vi "Dresden R2R Sputter 03.02.2018 IY24.vi"() -> ()   [LabVIEW 2009] (continued)
        n23727 = local write "R Single DC Step4 Coating Power"(w29188) -> ()
        n23728 = local write "R Single RF Step2 Coating Power"(w29146) -> ()
        n23729 = local write "R Single RF Interval length"(w29148) -> ()
        n23730 = case shown="2" w29281 {
          frame #0 {
          }
          frame #1 {
            n23731 = local write "R_Recipe_type_selection"(enum32{"Single Recipe", "Combination Sputter"}."Single Recipe" ("R_Recipe_type_selection")) -> ()
          }
          frame #2 {
            n23732 = local write "R_Recipe_type_selection"(enum32{"Single Recipe", "Combination Sputter"}."Combination Sputter" ("R_Recipe_type_selection")) -> ()
          }
        }
        n23733 = local write "R Single RF Step3 Coating Power"(w29144) -> ()
        n23734 = local write "R Web speed(cm/min)"(w29259) -> ()
        n23735 = Boolean Array To Number(Boolean array=w29296) -> (number=w29295:u32)
        n23736 = local write "R Single RF Step4 Coating Power"(w29142) -> ()
        n23737 = local write "R Maximum diameter"(w29261) -> ()
        n23738 = case shown="2" w29348 {
          frame #0 {
          }
          frame #1 {
            n23739 = local write "R_Web_selection"(enum32{"Web", "Other"}."Web" ("R_Web_selection")) -> ()
          }
          frame #2 {
            n23740 = local write "R_Web_selection"(enum32{"Web", "Other"}."Other" ("R_Web_selection")) -> ()
          }
        }
        n23741 = local write "R Minimum diameter"(w29262) -> ()
        n23742 = local write "R_Single Microwave Power"(w28900) -> ()
        n23743 = local write "R Single RF Step5 Coating Power"(w29138) -> ()
        n23744 = local write "R_Single Microwave Time"(w29233) -> ()
        n23745 = local write "R Single Microwave Number"(w29234) -> ()
        n23746 = local write "R _Total_length"(w28935) -> ()
        n23747 = Mantissa & Exponent(0:w29295) -> (2:w29289:dbl)  [unwired: 1 out]
        n23748 = local write "R Tension Value"(w29258) -> ()
        n23749 = local write "R Single RF Ramp down Time"(w29134) -> ()
        n23750 = local write "R Web thicness"(w29260) -> ()
        n23751 = case shown="2" w29300 {
          frame #0 {
          }
          frame #1 {
            n23752 = local write "R_Thickness Selection"(enum32{"Thickness", "Time"}."Thickness" ("R_Thickness Selection")) -> ()
          }
          frame #2 {
            n23753 = local write "R_Thickness Selection"(enum32{"Thickness", "Time"}."Time" ("R_Thickness Selection")) -> ()
          }
        }
        n23754 = case shown="3" w29289 {
          frame #0 {
          }
          frame #1 {
            n23755 = local write "R_Simple_Coating Type Selection"(T3."Microwave Plasma" ("R_Coating Type Selection")) -> ()
          }
          frame #2 {
            n23756 = local write "R_Simple_Coating Type Selection"(T3."DC Sputter" ("R_Coating Type Selection")) -> ()
          }
          frame #3 {
            n23757 = local write "R_Simple_Coating Type Selection"(T3."RF Sputter" ("R_Coating Type Selection")) -> ()
          }
        }
        n23758 = Build Array(FALSE, w28934, w28927) -> (w28931:bool[])
        n23759 = Boolean Array To Number(Boolean array=w28931) -> (number=w28932:u32)
        n23760 = Mantissa & Exponent(0:w28932) -> (2:w28929:dbl)  [unwired: 1 out]
        n23761 = stacked-sequence {
          frame #0 {
            # "Recipe Parameters"
          }
        }
        n23762 = case shown="1" w28929 {
          frame #0 {
          }
          frame #1 {
            n23763 = local write "R_DC_Chamber_selection"(enum32{"Chamber II", "Chamber III"}."Chamber II" ("R_DC_Chamber_selection")) -> ()
          }
          frame #2 {
            n23764 = local write "R_DC_Chamber_selection"(enum32{"Chamber II", "Chamber III"}."Chamber III" ("R_DC_Chamber_selection")) -> ()
          }
        }
      }
    }
    n23765 = case shown="True" "Edit_recipe" {
      frame #0 {
      }
      frame #1 {
        n23766 = call "Dresden Edit Recipe(in).vi"() -> ()  [unwired: 1 in]
      }
    }
    n23767 = case shown="True" "Edit_coating" {
      frame #0 {
      }
      frame #1 {
        n23768 = call "VK-1701Edit Coating.vi"() -> ()  [unwired: 3 in]
      }
    }
    n23769 = case shown="True" "New_recipe" {
      frame #0 {
      }
      frame #1 {
        n23770 = call "Dresden New Recipe(in).vi"() -> ()  [unwired: 2 out]
      }
    }
    n23771 = case shown="True" "New_coating" {
      frame #0 {
      }
      frame #1 {
        n23772 = call "VK-1701New Coating.vi"() -> ()  [unwired: 1 in, 2 out]
      }
    }
    n23773 = case shown="True" "Load_coating" {
      frame #0 {
      }
      frame #1 {
        n23774 = call "VK-1701Load Coating.vi"() -> ("Path Array"=w28844:string[])  [unwired: 1 in, 2 out]
        "Path Array" <- w28844
        n23775 = Array Size(array=w28844) -> (size(s)=w28847:i32)
        n23776 = Increment(x=w28847) -> (x+1=w28848:i32)
        n23777 = Reshape Array(w28844, w28848, w28848) -> (w28849:string[][])
        n23778 = Decrement(x=w28847) -> (x-1=→"Size":i32)
        n23779 = Transpose 2D Array(2D array=w28849) -> (transposed array=w28845:string[][])
        n23780 = property on="Recipe List" class="MCListbox (strict)"("ItemNames"=w28845) -> ()  [unwired: 2 in, 2 out]
      }
    }
    n23781 = local read "Start_coating"() -> (w28837:bool)
    n23782 = case shown="True" w28837 {
      frame #0 {
      }
      frame #1 {
        n23783 = local read "Semi"() -> (w28858:bool)
        n23784 = local read "Recipe_number"() -> (w28851:i32)
        n23785 = local read "Size"() -> (w28855:i32)
        n23786 = Or(x=w28858, y="Coat_int") -> (x .or. y?=w28861:bool)
        n23787 = Increment(x=w28855) -> (x+1=w28856:i32)
        n23788 = feedback #446() -> (w28852:i32)  [unwired: 1 in]
        n23789 = Equal?(x=w28851, y=w28856) -> (x = y?=w28857:bool)
        n23790 = Greater?(x=w28851, y=w28852) -> (0:w28853:bool)
        n23791 = Or(x=w28853, y=w28857) -> (x .or. y?=w28850:bool)
        n23792 = Build Array(FALSE, w28861, w28850) -> (w28863:bool[])
        n23793 = Boolean Array To Number(Boolean array=w28863) -> (number=w28862:u32)
        n23794 = Mantissa & Exponent(0:w28862) -> (2:w28854:dbl)  [unwired: 1 out]
        n23795 = case shown="2" w28854 {
          frame #0 {
            n23796 = stacked-sequence {
              tunnel: [w28870] -> w28864
              frame #0 {
                n23797 = local read "Recipe_number"() -> (w28872:i32)
                n23798 = local read "Size"() -> (w28873:i32)
                n23799 = Increment(x=w28873) -> (x+1=w28871:i32)
                n23800 = Equal?(x=w28872, y=w28871) -> (x = y?=w28870:bool)
              }
            }
            n23801 = case shown="False" w28864 {
              frame #0 {
                n23802 = property on="Recipe List" class="MCListbox (strict)"() -> ("ItemNames"=w28866:string[][])  [unwired: 2 in, 2 out]
                n23803 = local read "Recipe_number"() -> (w28867:i32)
                n23804 = Replace Array Subset(array=w28866, new element="Running" ("new element/subarray"), index (row)=w28867, index (col)=1 ("Column")) -> (w28865:string[][])
                n23805 = property on="Recipe List" class="MCListbox (strict)"("ItemNames"=w28865) -> ()  [unwired: 2 in, 2 out]
              }
              frame #1 {
              }
            }
          }
          frame #1 {
            n23806 = local read "Recipe_number"() -> (w28874:i32)
            n23807 = property on="Recipe List" class="MCListbox (strict)"() -> ("ItemNames"=w28876:string[][])  [unwired: 2 in, 2 out]
            n23808 = Replace Array Subset(array=w28876, new element="Not Completed !" ("new element/subarray"), index (row)=w28874, index (col)=1 ("Column")) -> (w28875:string[][])
            n23809 = property on="Recipe List" class="MCListbox (strict)"("ItemNames"=w28875) -> ()  [unwired: 2 in, 2 out]
          }
          frame #2 {
            n23810 = property on="Recipe List" class="MCListbox (strict)"() -> ("ItemNames"=w28880:string[][])  [unwired: 2 in, 2 out]
            n23811 = stacked-sequence {
              tunnel: [_ w28890] -> w28884
              frame #0 {
                n23812 = Wait (ms)(milliseconds to wait=u32 1000) -> ()  [unwired: 1 out]
              }
              frame #1 {
                n23813 = local read "Size"() -> (w28893:i32)
                n23814 = Less?(x=w28893, y=1) -> (x < y?=w28895:bool)
                n23815 = case shown="True" w28895 {
                  tunnel: [w28897 w28898] -> w28891
                  tunnel: w28893 -> [w28896 w28898]
                  frame #0 {
                    n23816 = Increment(x=w28896) -> (x+1=w28897:i32)
                  }
                  frame #1 {
                  }
                }
                n23817 = local read "Recipe_number"() -> (w28892:i32)
                n23818 = Equal?(x=w28892, y=w28891) -> (x = y?=w28890:bool)
              }
            }
            n23819 = case shown="False" w28884 {
              tunnel: [w28885 w28887] -> w28881
              frame #0 {
                n23820 = local read "Recipe_number"() -> (w28886:i32)
                n23821 = Decrement(x=w28886) -> (x-1=w28885:i32)
              }
              frame #1 {
                n23822 = local read "Recipe_number"() -> (w28888:i32)
                n23823 = Decrement(x=w28888) -> (x-1=w28887:i32)
              }
            }
            n23824 = Replace Array Subset(array=w28880, new element="Done" ("new element/subarray"), index (row)=w28881, index (col)=1 ("Column")) -> (w28879:string[][])
            n23825 = property on="Recipe List" class="MCListbox (strict)"("ItemNames"=w28879) -> ()  [unwired: 2 in, 2 out]
          }
        }
      }
    }
  }
  n23826 = while {
    stop <- FALSE stop-if-true
    n23827 = Wait Until Next ms Multiple(millisecond multiple=u32 300) -> ()  [unwired: 1 out]
    n23828 = Compound Arithmetic op=OR("Start_Coating_MW", "Start_Coating_Ch2", "Start_Coating_Ch3", "Start_Coating_Ch4") -> (w29415:bool)
    n23829 = case shown="True" w29415 {
      frame #0 {
      }
      frame #1 {
        n23830 = local write "Start_coating"(TRUE ("Start_coating")) -> ()
      }
    }
  }
  n23831 = while {
    stop <- FALSE stop-if-true
    n23832 = Wait Until Next ms Multiple(millisecond multiple=u32 300) -> ()  [unwired: 1 out]
    n23833 = case shown="True" "Start_coating" {
      frame #0 {
      }
      frame #1 {
        n23834 = while {
          i -> [w29428]
          stop <- w29422 stop-if-true
          n23835 = Wait Until Next ms Multiple(millisecond multiple=u32 300) -> ()  [unwired: 1 out]
          n23836 = local read "Path Array"() -> (w29427:string[])
          n23837 = Index Array(array=w29427, index=w29428) -> (element=w29425:string)
          "Path" <- w29425
          n23838 = Not Equal?(x="", y=w29425) -> (x != y?=w29424:bool)
          n23839 = case shown="True" w29424 {
            tunnel: [TRUE w29431] -> w29422
            frame #0 {
              w29429 = FALSE
              n23840 = local write "Start_Coating_MW"(w29429) -> ()
              n23841 = local write "Start_coating"(w29429) -> ()
              n23842 = local write "Start_Coating_Ch2"(w29429) -> ()
              n23843 = local write "Start_Coating_Ch3"(w29429) -> ()
              n23844 = local write "Start_Coating_Ch4"(w29429) -> ()
            }
            frame #1 {
              n23845 = stacked-sequence {
                tunnel: [FALSE _] -> w29431
                frame #0 {
                  # "All Recipe Parameters close &set zero"
                  n23846 = stacked-sequence {
                    frame #0 {
                      w29435 = FALSE ("Single_ Target_clean_cancel")
                      w29436 = FALSE ("Visible")
                      w29434 = TRUE ("Clean_MW_Coating")
                      w29437 = FALSE ("Cnt_Right_limit_do")
                      w29440 = FALSE ("R Single RF Ramp down")
                      w29441 = FALSE ("R Cmb Ch3 DC Target Clean Power Active")
                      w29442 = 0.0 ("R Cmb Ch2 Step4 Coating Power")
                      w29438 = 0.0 ("Preheating Temperature")
                      w29439 = "" ("Recipe Name :")
                      n23847 = local write "Substrate Material"(w29439) -> ()
                      n23848 = local write "R Cmb Ch2 Target material"(w29439) -> ()
                      n23849 = local write "R Single DC Target material"(w29439) -> ()
                      n23850 = local write "R Cmb Ch3 Target material"(w29439) -> ()
                      n23851 = local write "R Single RF Target material"(w29439) -> ()
                      n23852 = local write "Recipe Name"(w29439) -> ()
                      n23853 = property on="Process_tab_sputter 3" class="TabCtl (strict)"("Visible"=w29436) -> ()  [unwired: 2 in, 2 out]
                      n23854 = property on="Sputter_tab 3" class="TabCtl (strict)"("Visible"=w29436) -> ()  [unwired: 2 in, 2 out]
                      n23855 = property on="Process_tab_sputter" class="TabCtl (strict)"("Visible"=w29436) -> ()  [unwired: 2 in, 2 out]
                      n23856 = property on="Sputter_tab" class="TabCtl (strict)"("Visible"=w29436) -> ()  [unwired: 2 in, 2 out]
                      n23857 = property on="Sputter_tab 2" class="TabCtl (strict)"("Visible"=w29436) -> ()  [unwired: 2 in, 2 out]
                      n23858 = local write "R_Single Microwave Power"(w29438) -> ()
                      n23859 = local write "R_Single Microwave Time"(w29438) -> ()
                      n23860 = local write "R Single DC Ignition Power"(w29438) -> ()
                      n23861 = local write "R Single DC Target Clean Power"(w29438) -> ()
                      n23862 = local write "R Single DC Target Clean Time"(w29438) -> ()
                      n23863 = local write "R Single RF Ramp up Time"(w29438) -> ()
                      n23864 = local write "R Single RF Ignition Power"(w29438) -> ()
                      n23865 = local write "R Single RF Target Clean Power"(w29438) -> ()
                      n23866 = local write "R Single RF Target Clean Time"(w29438) -> ()
                      n23867 = local write "R Single RF Ramp down Time"(w29438) -> ()
                      n23868 = local write "R Cmb Ch2 DC Ignition Power"(w29438) -> ()
                      n23869 = local write "R Cmb Ch2 DC Target Clean Power"(w29438) -> ()
                      n23870 = local write "R Cmb Ch2 DC Target Clean Time"(w29438) -> ()
                      n23871 = local write "R Cmb Ch2 Step1 Coating Power"(w29438) -> ()
                      n23872 = local write "R Cmb Ch2 Step2 Coating Power"(w29438) -> ()
                      n23873 = local write "R Cmb Ch2 Step3 Coating Power"(w29438) -> ()
                      n23874 = local write "R _Total_length"(w29438) -> ()
                      n23875 = local write "R _Total_length"(w29438) -> ()
                      n23876 = local write "R Maximum diameter"(w29438) -> ()
                      n23877 = local write "R Minimum diameter"(w29438) -> ()
                      n23878 = local write "R Web thicness"(w29438) -> ()
                      n23879 = local write "R Web speed(cm/min)"(w29438) -> ()
                      n23880 = local write "R Tension Value"(w29438) -> ()
                      n23881 = local write "R Cmb Ch2 Step4 Coating Power"(w29442) -> ()
                      n23882 = local write "R Cmb Ch2 Step5 Coating Power"(w29442) -> ()
                      n23883 = local write "R Cmb Ch3 DC Ignition Power"(w29442) -> ()
                      n23884 = local write "R Cmb Ch3 DC Target Clean Power"(w29442) -> ()
                      n23885 = local write "R Cmb Ch3 DC Target Clean Time"(w29442) -> ()
                      n23886 = local write "R Cmb Ch3 Step1 Coating Power"(w29442) -> ()
                      n23887 = local write "R Cmb Ch3 Step2 Coating Power"(w29442) -> ()
                      n23888 = local write "R Cmb Ch3 Step3 Coating Power"(w29442) -> ()
                      n23889 = local write "R Cmb Ch3 Step4 Coating Power"(w29442) -> ()
                      n23890 = local write "R Cmb Ch3 Step5 Coating Power"(w29442) -> ()
                      n23891 = local write "R Single DC Step1 Coating Power"(w29442) -> ()
                      n23892 = local write "R Single DC Step2 Coating Power"(w29442) -> ()
                      n23893 = local write "R Single DC Step3 Coating Power"(w29442) -> ()
                      n23894 = local write "R Single DC Step4 Coating Power"(w29442) -> ()
                      n23895 = local write "R Single DC Step5 Coating Power"(w29442) -> ()
                      n23896 = local write "R Single RF  Step1 Coating Power"(w29442) -> ()
                      n23897 = local write "R Single RF Step2 Coating Power"(w29442) -> ()
                      n23898 = local write "R Single RF Step3 Coating Power"(w29442) -> ()
                      n23899 = local write "R Single RF Step4 Coating Power"(w29442) -> ()
                      n23900 = local write "R Single RF Step5 Coating Power"(w29442) -> ()
                      n23901 = local write "R Single Microwave Number"(w29442) -> ()
                      n23902 = local write "R Single RF Target Clean"(w29441) -> ()
                      n23903 = local write "R Cmb Ch3 DC Target Clean Power Active"(w29441) -> ()
                      n23904 = local write "R Cmb Ch3 Material ok"(w29441) -> ()
                      n23905 = local write "R Cmb Ch2 Step5 Coating Power Active"(w29441) -> ()
                      n23906 = local write "R Cmb Ch2 Step4 Coating Power Active"(w29441) -> ()
                      n23907 = local write "R Cmb Ch2 Step3 Coating Power Active"(w29441) -> ()
                      n23908 = local write "R Cmb Ch2 Step2 Coating Power Active"(w29441) -> ()
                      n23909 = local write "R Cmb Ch2 Step1 Coating Power Active"(w29441) -> ()
                      n23910 = local write "R Cmb Ch2 DC Target Clean Power Active"(w29441) -> ()
                      n23911 = local write "R_Cmb Ch2_Material ok"(w29441) -> ()
                      n23912 = local write "R_Single DC_Material ok"(w29441) -> ()
                      n23913 = local write "R Single DC Target Clean"(w29441) -> ()
                      n23914 = local write "R_Single RF Material ok"(w29441) -> ()
                      n23915 = local write "R Single RF Ramp up"(w29441) -> ()
                      n23916 = Wait (ms)(milliseconds to wait=u32 2000) -> ()  [unwired: 1 out]
                      n23917 = local write "R Single RF Ramp down"(w29440) -> ()
                      n23918 = local write "Thickness_Monitor_Active"(w29440) -> ()
                      n23919 = local write "R Single DC Step1 Coating Power Active"(w29440) -> ()
                      n23920 = local write "R Single DC Step2 Coating Power Active"(w29440) -> ()
                      n23921 = local write "R Single DC Step3 Coating Power Active"(w29440) -> ()
                      n23922 = local write "R Single DC Step4 Coating Power Active"(w29440) -> ()
                      n23923 = local write "R Single DC Step5 Coating Power Active"(w29440) -> ()
                      n23924 = local write "R Single RF Step1 Coating Power Active"(w29440) -> ()
                      n23925 = local write "R Single RF Step2 Coating Power Active"(w29440) -> ()
                      n23926 = local write "R Single RF Step4 Coating Power Active"(w29440) -> ()
                      n23927 = local write "R Single RF Step5 Coating Power Active"(w29440) -> ()
                      n23928 = local write "R Single RF Step3 Coating Power Active"(w29440) -> ()
                      n23929 = local write "Sputter_cancel"(w29435) -> ()
                      n23930 = local write "Sputter_cancel 2"(w29435) -> ()
                      n23931 = local write "Sputter_cancel 3"(w29435) -> ()
                      n23932 = local write "Abort_sputter"(w29435) -> ()
                      n23933 = local write "Abort_sputter 2"(w29435) -> ()
                      n23934 = local write "Abort_sputter 3"(w29435) -> ()
                      n23935 = local write "Cnt_Right_limit_do"(w29437) -> ()
                      n23936 = local write "Cnt_Right_slow_do"(w29437) -> ()
                      n23937 = local write "Cnt_Left_slow_do"(w29437) -> ()
                      n23938 = local write "Cnt_Left_limit_do"(w29437) -> ()
                      n23939 = local write "Clean_MW_Coating"(w29434) -> ()
                      n23940 = local write "Clean_Single_DC1"(w29434) -> ()
                      n23941 = local write "Clean_Single_DC2"(w29434) -> ()
                      n23942 = local write "Clean_Single_RF"(w29434) -> ()
                      n23943 = local write "Clean_Combo"(w29434) -> ()
                    }
                    frame #1 {
                      w29443 = FALSE ("Ch1_mw_active")
                      n23944 = local write "Ch1_mw_active"(w29443) -> ()
                      n23945 = local write "Ch2_dc_active"(w29443) -> ()
                      n23946 = local write "Ch3_dc_active"(w29443) -> ()
                      n23947 = local write "Ch4_rf_active"(w29443) -> ()
                      n23948 = Wait (ms)(milliseconds to wait=u32 500) -> ()  [unwired: 1 out]
                    }
                  }
                }
                frame #1 {
                  n23949 = local read "R_Recipe_type_selection"() -> (w29445:enum32{"Single Recipe", "Combination Sputter"})
                  n23950 = case shown="\"Combination Sputter\"" w29445 {
                    frame #0 {
                      n23951 = local read "R_Simple_Coating Type Selection"() -> (w29446:T3)
                      n23952 = case shown="\"RF Sputter\"" w29446 {
                        frame #0 {
                          n23953 = local read "Ch1_pressure"() -> (w29451:dbl)
                          n23954 = local read "started_up_ch1"() -> (w29447:bool)
                          n23955 = In Range and Coerce(upper limit="MW_Coating_Interlock", x=w29451, lower limit=1e-08) -> (In Range?=w29452:bool)  [unwired: 1 out]
                          n23956 = And(x=w29452, y=w29447) -> (x .and. y?=w29448:bool)
                          n23957 = case shown="True" w29448 {
                            frame #0 {
                            }
                            frame #1 {
                              n23958 = local read "Semi"() -> (w29453:bool)
                              n23959 = case shown="False" w29453 {
                                frame #0 {
                                n23960 = stacked-sequence {
                                frame #0 {
                                n23961 = stacked-sequence {
                                frame #0 {
                                n23962 = local read "Semi"() -> (w29454:bool)
                                n23963 = case shown="False" w29454 {
                                frame #0 {
                                w29457 = FALSE ("Casette_servo_start/stop_do")
                                n23964 = local write "Ch1_Sov_Ar_do"(FALSE ("Ch1_Sov_Ar_do")) -> ()
                                n23965 = local write "Ar_auto_set_zero_ch1"(TRUE ("Dc_auto_set_zero")) -> ()
                                n23966 = local write "MW1_off"(TRUE ("MW1_off")) -> ()
                                n23967 = local write "final_process_messages"("Coating was Completed" ("final_process_messages")) -> ()
                                n23968 = local write "system_status"("Coating Mode is Active" ("system_status")) -> ()
                                n23969 = local write "Casette_servo_start/stop_do"(w29457) -> ()
                                n23970 = local write "Tension_controllers_start/stop_do"(w29457) -> ()
                                }
                                frame #1 {
                                }
                                }
                                }
                                frame #1 {
                                n23971 = local read "Semi"() -> (w29461:bool)
                                n23972 = case shown="False" w29461 {
                                frame #0 {
                                n23973 = Wait (ms)(milliseconds to wait=u32 2500) -> ()  [unwired: 1 out]
                                }
                                frame #1 {
                                }
                                }
                                }
                                frame #2 {
                                n23974 = local read "Semi"() -> (w29463:bool)
                                n23975 = case shown="False" w29463 {
                                frame #0 {
                                n23976 = local write "Ch1_SRV_start_stop_do"(FALSE ("Ch1_SRV_start_stop_do")) -> ()
                                n23977 = local write "MW2_off"(FALSE ("MW1_off")) -> ()
                                }
                                frame #1 {
                                }
                                }
                                }
                                frame #3 {
                                n23978 = local read "Semi"() -> (w29466:bool)
                                n23979 = case shown="False" w29466 {
                                frame #0 {
                                n23980 = Wait (ms)(milliseconds to wait=u32 2500) -> ()  [unwired: 1 out]
                                }
                                frame #1 {
                                }
                                }
                                }
                                frame #4 {
                                n23981 = local read "Semi"() -> (w29468:bool)
                                n23982 = case shown="False" w29468 {
                                frame #0 {
                                n23983 = local write "SMW1"(TRUE ("CMW1")) -> ()
                                n23984 = Wait (ms)(milliseconds to wait=u32 1000) -> ()  [unwired: 1 out]
                                }
                                frame #1 {
                                }
                                }
                                }
                                }
                                }
                                frame #1 {
                                n23985 = local read "ch_present_position"() -> (w29472:dbl)
                                n23986 = Not Equal?(x=w29472, y=1.0) -> (x != y?=w29473:bool)
                                n23987 = case shown="True" w29473 {
                                frame #0 {
                                }
                                frame #1 {
                                n23988 = stacked-sequence {
                                frame #0 {
                                n23989 = local write "Set chamber"(1.0 ("Set chamber")) -> ()
                                n23990 = Wait (ms)(milliseconds to wait=u32 100) -> ()  [unwired: 1 out]
                                }
                                frame #1 {
                                n23991 = local write "Auto_set_transfer"(TRUE ("Auto_set_transfer")) -> ()
                                }
                                frame #2 {
                                n23992 = while {
                                stop <- w29478 stop-if-true
                                n23993 = Wait Until Next ms Multiple(millisecond multiple=u32 300) -> ()  [unwired: 1 out]
                                n23994 = local read "Auto_set_transfer"() -> (w29479:bool)
                                n23995 = local read "Semi"() -> (w29481:bool)
                                n23996 = Not(x=w29479) -> (.not. x?=w29480:bool)
                                n23997 = Or(x=w29480, y=w29481) -> (x .or. y?=w29478:bool)
                                }
                                }
                                frame #3 {
                                n23998 = local write "SMW1 2"(TRUE ("SMW1 2")) -> ()
                                n23999 = Wait (ms)(milliseconds to wait=u32 300) -> ()  [unwired: 1 out]
                                }
                                }
                                }
                                }
                                }
                                frame #2 {
                                # "WATER FLOW CONTROL OPEN"
                                n24000 = stacked-sequence {
                                frame #0 {
                                n24001 = local read "Semi"() -> (w29484:bool)
                                n24002 = case shown="False" w29484 {
                                frame #0 {
                                n24003 = while {
                                i -> [w29490]
                                stop <- w29485 stop-if-true
                                n24004 = Greater?(x=w29490, y=100) -> (0:w29489:bool)
                                n24005 = case shown="True" w29489 {
                                frame #0 {
                                }
                                frame #1 {
                                n24006 = local write "Semi"(TRUE ("Semi")) -> ()
                                n24007 = local write "Error Message"("Coating Process  \nwas cancelled.\nPlease check water \nflow connection." ("Error Message")) -> ()
                                }
                                }
                                n24008 = local read "Ch4_WFS_di"() -> (w29488:bool)
                                n24009 = case shown="True" w29488 {
                                tunnel: [TRUE FALSE] -> w29487
                                frame #0 {
                                }
                                frame #1 {
                                n24010 = local write "Ch4_WFC_do"(FALSE ("Ch1_WFC_do")) -> ()
                                n24011 = Wait Until Next ms Multiple(millisecond multiple=u32 200) -> ()  [unwired: 1 out]
                                }
                                }
                                n24012 = local read "Semi"() -> (w29486:bool)
                                n24013 = Or(x=w29487, y=w29486) -> (x .or. y?=w29485:bool)
                                }
                                }
                                frame #1 {
                                }
                                }
                                }
                                frame #1 {
                                n24014 = local read "Semi"() -> (w29498:bool)
                                n24015 = case shown="False" w29498 {
                                frame #0 {
                                n24016 = while {
                                i -> [w29504]
                                stop <- w29499 stop-if-true
                                n24017 = Greater?(x=w29504, y=100) -> (0:w29503:bool)
                                n24018 = case shown="True" w29503 {
                                frame #0 {
                                }
                                frame #1 {
                                n24019 = local write "Semi"(TRUE ("Semi")) -> ()
                                n24020 = local write "Error Message"("Coating Process  \nwas cancelled.\nPlease check water \nflow connection." ("Error Message")) -> ()
                                }
                                }
                                n24021 = local read "Ch3_WFS_di"() -> (w29502:bool)
                                n24022 = case shown="True" w29502 {
                                tunnel: [TRUE FALSE] -> w29501
                                frame #0 {
                                }
                                frame #1 {
                                n24023 = local write "Ch3_WFC_do"(FALSE ("Ch1_WFC_do")) -> ()
                                n24024 = Wait Until Next ms Multiple(millisecond multiple=u32 200) -> ()  [unwired: 1 out]
                                }
                                }
                                n24025 = local read "Semi"() -> (w29500:bool)
                                n24026 = Or(x=w29501, y=w29500) -> (x .or. y?=w29499:bool)
                                }
                                }
                                frame #1 {
                                }
                                }
                                }
                                frame #2 {
                                n24027 = local read "Semi"() -> (w29512:bool)
                                n24028 = case shown="False" w29512 {
                                frame #0 {
                                n24029 = while {
                                i -> [w29518]
                                stop <- w29513 stop-if-true
                                n24030 = Greater?(x=w29518, y=100) -> (0:w29517:bool)
                                n24031 = case shown="True" w29517 {
                                frame #0 {
                                }
                                frame #1 {
                                n24032 = local write "Semi"(TRUE ("Semi")) -> ()
                                n24033 = local write "Error Message"("Coating Process  \nwas cancelled.\nPlease check water \nflow connection." ("Error Message")) -> ()
                                }
                                }
                                n24034 = local read "Ch2_WFS_di"() -> (w29516:bool)
                                n24035 = case shown="True" w29516 {
                                tunnel: [TRUE FALSE] -> w29515
                                frame #0 {
                                }
                                frame #1 {
                                n24036 = local write "Ch2_WFC_do"(FALSE ("Ch1_WFC_do")) -> ()
                                n24037 = Wait Until Next ms Multiple(millisecond multiple=u32 200) -> ()  [unwired: 1 out]
                                }
                                }
                                n24038 = local read "Semi"() -> (w29514:bool)
                                n24039 = Or(x=w29515, y=w29514) -> (x .or. y?=w29513:bool)
                                }
                                }
                                frame #1 {
                                }
                                }
                                }
                                frame #3 {
                                n24040 = local read "Semi"() -> (w29526:bool)
                                n24041 = case shown="False" w29526 {
                                frame #0 {
                                n24042 = while {
                                i -> [w29532]
                                stop <- w29527 stop-if-true
                                n24043 = Greater?(x=w29532, y=100) -> (0:w29531:bool)
                                n24044 = case shown="True" w29531 {
                                frame #0 {
                                }
                                frame #1 {
                                n24045 = local write "Semi"(TRUE ("Semi")) -> ()
                                n24046 = local write "Error Message"("Coating Process  \nwas cancelled.\nPlease check water \nflow connection." ("Error Message")) -> ()
                                }
                                }
                                n24047 = local read "Ch1_WFS_di"() -> (w29530:bool)
                                n24048 = case shown="False" w29530 {
                                tunnel: [FALSE TRUE] -> w29529
                                frame #0 {
                                n24049 = local write "Ch1_WFC_do"(TRUE ("Ch1_WFC_do")) -> ()
                                n24050 = Wait Until Next ms Multiple(millisecond multiple=u32 200) -> ()  [unwired: 1 out]
                                }
                                frame #1 {
                                }
                                }
                                n24051 = local read "Semi"() -> (w29528:bool)
                                n24052 = Or(x=w29529, y=w29528) -> (x .or. y?=w29527:bool)
                                }
                                }
                                frame #1 {
                                }
                                }
                                }
                                frame #4 {
                                n24053 = local read "Semi"() -> (w29540:bool)
                                n24054 = case shown="False" w29540 {
                                frame #0 {
                                n24055 = local write "SMW2"(TRUE ("CMW2")) -> ()
                                n24056 = Wait (ms)(milliseconds to wait=u32 1000) -> ()  [unwired: 1 out]
                                }
                                frame #1 {
                                }
                                }
                                }
                                }
                                }
                                frame #3 {
                                # "CC CLOSE"
                                n24057 = stacked-sequence {
                                frame #0 {
                                n24058 = local read "Semi"() -> (w29543:bool)
                                n24059 = case shown="False" w29543 {
                                frame #0 {
                                n24060 = while {
                                i -> [w29549]
                                stop <- w29544 stop-if-true
                                n24061 = Greater?(x=w29549, y=50) -> (0:w29548:bool)
                                n24062 = case shown="True" w29548 {
                                frame #0 {
                                }
                                frame #1 {
                                n24063 = local write "Semi"(TRUE ("Semi")) -> ()
                                n24064 = local write "Error Message"("Coating Process  \nwas cancelled.\nPlease check \nBG-BV connection." ("Error Message")) -> ()
                                }
                                }
                                n24065 = local read "Ch1_Cc_on_off_di"() -> (w29547:bool)
                                n24066 = case shown="True" w29547 {
                                tunnel: [TRUE FALSE] -> w29546
                                frame #0 {
                                }
                                frame #1 {
                                n24067 = local write "Ch1_Cc_on_off_do"(FALSE ("Ch1_WFC_do")) -> ()
                                n24068 = Wait Until Next ms Multiple(millisecond multiple=u32 200) -> ()  [unwired: 1 out]
                                }
                                }
                                n24069 = local read "Semi"() -> (w29545:bool)
                                n24070 = Or(x=w29546, y=w29545) -> (x .or. y?=w29544:bool)
                                }
                                }
                                frame #1 {
                                }
                                }
                                }
                                frame #1 {
                                n24071 = local read "Semi"() -> (w29557:bool)
                                n24072 = case shown="False" w29557 {
                                frame #0 {
                                n24073 = local write "SMW3"(TRUE ("CMW2")) -> ()
                                n24074 = Wait (ms)(milliseconds to wait=u32 1000) -> ()  [unwired: 1 out]
                                }
                                frame #1 {
                                }
                                }
                                }
                                }
                                }
                                frame #4 {
                                # "BG-BV close"
                                n24075 = stacked-sequence {
                                frame #0 {
                                n24076 = local read "Semi"() -> (w29560:bool)
                                n24077 = case shown="False" w29560 {
                                frame #0 {
                                n24078 = while {
                                i -> [w29566]
                                stop <- w29561 stop-if-true
                                n24079 = Greater?(x=w29566, y=50) -> (0:w29565:bool)
                                n24080 = case shown="True" w29565 {
                                frame #0 {
                                }
                                frame #1 {
                                n24081 = local write "Semi"(TRUE ("Semi")) -> ()
                                n24082 = local write "Error Message"("Coating Process  \nwas cancelled.\nPlease check \nBG-BV connection." ("Error Message")) -> ()
                                }
                                }
                                n24083 = local read "Ch1_Bg_bv_di"() -> (w29564:bool)
                                n24084 = case shown="True" w29564 {
                                tunnel: [TRUE FALSE] -> w29563
                                frame #0 {
                                }
                                frame #1 {
                                n24085 = local write "Ch1_Bg_bv_do"(FALSE ("Ch1_WFC_do")) -> ()
                                n24086 = Wait Until Next ms Multiple(millisecond multiple=u32 200) -> ()  [unwired: 1 out]
                                }
                                }
                                n24087 = local read "Semi"() -> (w29562:bool)
                                n24088 = Or(x=w29563, y=w29562) -> (x .or. y?=w29561:bool)
                                }
                                }
                                frame #1 {
                                }
                                }
                                }
                                frame #1 {
                                n24089 = local read "Semi"() -> (w29574:bool)
                                n24090 = case shown="False" w29574 {
                                frame #0 {
                                n24091 = local write "SMW4"(TRUE ("CMW2")) -> ()
                                n24092 = Wait (ms)(milliseconds to wait=u32 1000) -> ()  [unwired: 1 out]
                                }
                                frame #1 {
                                }
                                }
                                }
                                }
                                }
                                frame #5 {
                                # "PC-BV CLOSE"
                                n24093 = stacked-sequence {
                                frame #0 {
                                n24094 = local read "Semi"() -> (w29577:bool)
                                n24095 = case shown="False" w29577 {
                                frame #0 {
                                n24096 = stacked-sequence {
                                frame #0 {
                                n24097 = local read "Semi"() -> (w29578:bool)
                                n24098 = case shown="False" w29578 {
                                frame #0 {
                                n24099 = local write "Pc_bv1_auto_close"(TRUE ("Tp1_auto_start")) -> ()
                                }
                                frame #1 {
                                }
                                }
                                }
                                frame #1 {
                                n24100 = local read "Semi"() -> (w29580:bool)
                                n24101 = case shown="False" w29580 {
                                frame #0 {
                                n24102 = Wait (ms)(milliseconds to wait=u32 1000) -> ()  [unwired: 1 out]
                                }
                                frame #1 {
                                }
                                }
                                }
                                frame #2 {
                                n24103 = local read "Semi"() -> (w29582:bool)
                                n24104 = case shown="False" w29582 {
                                frame #0 {
                                n24105 = while {
                                i -> [w29588]
                                stop <- w29584 stop-if-true
                                n24106 = local read "Pc_bv_closed_ch1"() -> (w29586:bool)
                                n24107 = Greater?(x=w29588, y=120) -> (0:w29587:bool)
                                n24108 = local read "Semi"() -> (w29585:bool)
                                n24109 = Compound Arithmetic op=OR(w29585, w29586, w29587) -> (w29584:bool)
                                n24110 = Wait (ms)(milliseconds to wait=u32 500) -> ()  [unwired: 1 out]
                                }